vi "HFRR ADV v044.vi"() -> ()   [LabVIEW 2025] (continued)
                "image data" <- w1507
                n1350 = local write "Print 3"(FALSE ("Print 2")) -> ()
                n1351 = call <vilib>:"Draw Flattened Pixmap.vi"("image data"=w1507) -> ("new picture"=→"new picture":picture)  [unwired: 8 in]
              }
              frame Error {
              }
            }
          }
        }
      }
    }
    n1352 = Wait (ms)(milliseconds to wait=u32 20 ("millisecond timer value")) -> ()  [unwired: 1 out]
    n1353 = local read "Quit"() -> (w1440:bool)
  }
  n1354 = while {
    tunnel: w43 -> [_]
    tunnel: w29 -> [_]
    stop <- w1537 stop-if-true
    # "New Adv Logics"
    n1355 = local read "Main Tab"() -> (w1518:T4)
    n1356 = local read "Main Tab"() -> (w1535:T4)
    n1357 = local read "Sign In"() -> (w1534:bool)
    n1358 = case shown="\"Adv Scar\"" w1518 {
      frame "HOME", Default {
        n1359 = local read "LIVE FEED MIN TEMP"() -> (w1670:bool)
        n1360 = local write "LIVE FEED MAX TEMP"(TRUE ("LIVE FEED MAX TEMP")) -> ()
        n1361 = local read "CAMERA ROI MIN TEMP"() -> (w1668:bool)
        n1362 = case shown="True" w1670 {
          selector: w1670 -> [_ w1677]
          frame False {
          }
          frame True {
            n1363 = Not(x=w1677) -> (.not. x?=w1676:bool)
            n1364 = local write "LIVE FEED MIN TEMP"(w1676) -> ()
            n1365 = call "CAMERA LIVE FEED FGV.vi"("Enum - Menu"=CAMERA_LIVE_FEED_ENUM."CAMERA MINIMIZE") -> ()  [unwired: 9 in, 2 out]
          }
        }
        n1366 = case shown="True" w1668 {
          selector: w1668 -> [_ w1674]
          frame False {
          }
          frame True {
            n1367 = Not(x=w1674) -> (.not. x?=w1673:bool)
            n1368 = local write "CAMERA ROI MIN TEMP"(w1673) -> ()
            n1369 = call "IMAGE ANALYSIS.vi"("Enum"=POST_ANALYSIS_ENUM."MINIMIZE UI") -> ()  [unwired: 9 in, 2 out]
          }
        }
        n1370 = local write "CAMERA ROI MAX TEMP"(TRUE ("CAMERA ROI MAX TEMP")) -> ()
      }
      frame "Test Setup" {
        n1371 = local read "LIVE FEED MIN TEMP"() -> (w1680:bool)
        n1372 = local read "CAMERA ROI MIN TEMP"() -> (w1678:bool)
        n1373 = local write "LIVE FEED MAX TEMP"(TRUE ("LIVE FEED MAX TEMP")) -> ()
        n1374 = case shown="True" w1680 {
          selector: w1680 -> [_ w1687]
          frame False {
          }
          frame True {
            n1375 = Not(x=w1687) -> (.not. x?=w1686:bool)
            n1376 = local write "LIVE FEED MIN TEMP"(w1686) -> ()
            n1377 = call "CAMERA LIVE FEED FGV.vi"("Enum - Menu"=CAMERA_LIVE_FEED_ENUM."CAMERA MINIMIZE") -> ()  [unwired: 9 in, 2 out]
          }
        }
        n1378 = case shown="True" w1678 {
          selector: w1678 -> [_ w1684]
          frame False {
          }
          frame True {
            n1379 = Not(x=w1684) -> (.not. x?=w1683:bool)
            n1380 = local write "CAMERA ROI MIN TEMP"(w1683) -> ()
            n1381 = call "IMAGE ANALYSIS.vi"("Enum"=POST_ANALYSIS_ENUM."MINIMIZE UI") -> ()  [unwired: 9 in, 2 out]
          }
        }
        n1382 = local write "CAMERA ROI MAX TEMP"(TRUE ("CAMERA ROI MAX TEMP")) -> ()
      }
      frame "Acquire" {
        n1383 = local read "LIVE FEED MIN TEMP"() -> (w1690:bool)
        n1384 = local write "LIVE FEED MAX TEMP"(TRUE ("LIVE FEED MAX TEMP")) -> ()
        n1385 = local read "CAMERA ROI MIN TEMP"() -> (w1688:bool)
        n1386 = case shown="True" w1690 {
          selector: w1690 -> [_ w1697]
          frame False {
          }
          frame True {
            n1387 = Not(x=w1697) -> (.not. x?=w1696:bool)
            n1388 = local write "LIVE FEED MIN TEMP"(w1696) -> ()
            n1389 = call "CAMERA LIVE FEED FGV.vi"("Enum - Menu"=CAMERA_LIVE_FEED_ENUM."CAMERA MINIMIZE") -> ()  [unwired: 9 in, 2 out]
          }
        }
        n1390 = case shown="True" w1688 {
          selector: w1688 -> [_ w1694]
          frame False {
          }
          frame True {
            n1391 = Not(x=w1694) -> (.not. x?=w1693:bool)
            n1392 = local write "CAMERA ROI MIN TEMP"(w1693) -> ()
            n1393 = call "IMAGE ANALYSIS.vi"("Enum"=POST_ANALYSIS_ENUM."MINIMIZE UI") -> ()  [unwired: 9 in, 2 out]
          }
        }
        n1394 = local write "CAMERA ROI MAX TEMP"(TRUE ("CAMERA ROI MAX TEMP")) -> ()
      }
      frame "Adv Scar" {
        n1395 = local read "CAMERA ROI MIN TEMP"() -> (w1698:bool)
        n1396 = case shown="True" "LIVE FEED MAX TEMP" {
          selector: "LIVE FEED MAX TEMP" -> [_ w1719]
          frame False {
          }
          frame True {
            n1397 = Not(x=w1719) -> (.not. x?=w1718:bool)
            n1398 = local write "LIVE FEED MAX TEMP"(w1718) -> ()
            n1399 = call "CAMERA LIVE FEED FGV.vi"("Enum - Menu"=CAMERA_LIVE_FEED_ENUM."CAMERA RESTORE") -> ("error out"=w1709:errorcluster)  [unwired: 9 in, 1 out]
            n1400 = Type Cast(type=30, x=0) -> (*(type *) &x=w1713:i32)
            n1401 = Add(x=w1713, y=48) -> (x+y=w1714:i32)
            n1402 = call "CAMERA LIVE FEED FGV.vi"("Enum - Menu"=CAMERA_LIVE_FEED_ENUM."CAMERA MODE SET", "error in (no error)"=w1709, "CAMERA MODE"=w1714) -> ("error out"=w1706:errorcluster)  [unwired: 7 in, 1 out]
            n1403 = call "CAMERA LIVE FEED FGV.vi"("Enum - Menu"=CAMERA_LIVE_FEED_ENUM."CAMERA GRAY", "error in (no error)"=w1706) -> ("error out"=w1705:errorcluster)  [unwired: 8 in, 1 out]
            n1404 = call "LIST FILE NAMES.vi"("error in (no error)"=w1705) -> ("error out"=w1715:errorcluster, "filenames"=w1716:string[])  [unwired: 9 in]
            n1405 = property on="FILE 3" class="CmbBox"(error in=w1715, "Strings[]"=w1716) -> ()  [unwired: 1 in, 2 out]
          }
        }
        n1406 = case shown="True" w1698 {
          selector: w1698 -> [_ w1704]
          frame False {
          }
          frame True {
            n1407 = Not(x=w1704) -> (.not. x?=w1703:bool)
            n1408 = local write "CAMERA ROI MIN TEMP"(w1703) -> ()
            n1409 = call "IMAGE ANALYSIS.vi"("Enum"=POST_ANALYSIS_ENUM."MINIMIZE UI") -> ()  [unwired: 9 in, 2 out]
          }
        }
        n1410 = local write "CAMERA ROI MAX TEMP"(TRUE ("CAMERA ROI MAX TEMP")) -> ()
        "LIVE FEED MIN TEMP" <- TRUE ("LIVE FEED MIN TEMP")
      }
      frame "Adv Scar Report" {
        n1411 = local read "CAMERA ROI MAX TEMP"() -> (w1720:bool)
        n1412 = local read "LIVE FEED MIN TEMP"() -> (w1722:bool)
        n1413 = local write "LIVE FEED MAX TEMP"(TRUE ("LIVE FEED MAX TEMP")) -> ()
        n1414 = case shown="True" w1722 {
          selector: w1722 -> [_ w1731]
          frame False {
          }
          frame True {
            n1415 = Not(x=w1731) -> (.not. x?=w1730:bool)
            n1416 = local write "LIVE FEED MIN TEMP"(w1730) -> ()
            n1417 = call "CAMERA LIVE FEED FGV.vi"("Enum - Menu"=CAMERA_LIVE_FEED_ENUM."CAMERA MINIMIZE") -> ()  [unwired: 9 in, 2 out]
          }
        }
        n1418 = case shown="True" w1720 {
          selector: w1720 -> [_ w1728]
          frame False {
          }
          frame True {
            n1419 = Not(x=w1728) -> (.not. x?=w1726:bool)
            n1420 = local write "CAMERA ROI MAX TEMP"(w1726) -> ()
            n1421 = call "IMAGE ANALYSIS.vi"("Enum"=POST_ANALYSIS_ENUM."SHOW UI") -> ("error out"=w1725:errorcluster)  [unwired: 9 in, 1 out]
            n1422 = call "LIST FILE NAMES.vi"("error in (no error)"=w1725) -> ("filenames"=w1724:string[])  [unwired: 9 in, 1 out]
            n1423 = property on="Test File List :" class="CmbBox"("Strings[]"=w1724) -> ()  [unwired: 2 in, 2 out]
          }
        }
        n1424 = local write "CAMERA ROI MIN TEMP"(TRUE ("CAMERA ROI MIN TEMP")) -> ()
      }
      frame "Compare Files" {
        n1425 = local read "LIVE FEED MIN TEMP"() -> (w1734:bool)
        n1426 = local write "LIVE FEED MAX TEMP"(TRUE ("LIVE FEED MAX TEMP")) -> ()
        n1427 = local read "CAMERA ROI MIN TEMP"() -> (w1732:bool)
        n1428 = case shown="True" w1734 {
          selector: w1734 -> [_ w1741]
          frame False {
          }
          frame True {
            n1429 = Not(x=w1741) -> (.not. x?=w1740:bool)
            n1430 = local write "LIVE FEED MIN TEMP"(w1740) -> ()
            n1431 = call "CAMERA LIVE FEED FGV.vi"("Enum - Menu"=CAMERA_LIVE_FEED_ENUM."CAMERA MINIMIZE") -> ()  [unwired: 9 in, 2 out]
          }
        }
        n1432 = case shown="True" w1732 {
          selector: w1732 -> [_ w1738]
          frame False {
          }
          frame True {
            n1433 = Not(x=w1738) -> (.not. x?=w1737:bool)
            n1434 = local write "CAMERA ROI MIN TEMP"(w1737) -> ()
            n1435 = call "IMAGE ANALYSIS.vi"("Enum"=POST_ANALYSIS_ENUM."MINIMIZE UI") -> ()  [unwired: 9 in, 2 out]
          }
        }
        n1436 = local write "CAMERA ROI MAX TEMP"(TRUE ("CAMERA ROI MAX TEMP")) -> ()
      }
      frame "About" {
        n1437 = local read "LIVE FEED MIN TEMP"() -> (w1744:bool)
        n1438 = local write "LIVE FEED MAX TEMP"(TRUE ("LIVE FEED MAX TEMP")) -> ()
        n1439 = local read "CAMERA ROI MIN TEMP"() -> (w1743:bool)
        n1440 = case shown="True" w1744 {
          selector: w1744 -> [_ w1751]
          frame False {
          }
          frame True {
            n1441 = Not(x=w1751) -> (.not. x?=w1750:bool)
            n1442 = local write "LIVE FEED MIN TEMP"(w1750) -> ()
            n1443 = call "CAMERA LIVE FEED FGV.vi"("Enum - Menu"=CAMERA_LIVE_FEED_ENUM."CAMERA MINIMIZE") -> ()  [unwired: 9 in, 2 out]
          }
        }
        n1444 = case shown="True" w1743 {
          selector: w1743 -> [_ w1748]
          frame False {
          }
          frame True {
            n1445 = Not(x=w1748) -> (.not. x?=w1747:bool)
            n1446 = local write "CAMERA ROI MIN TEMP"(w1747) -> ()
            n1447 = call "IMAGE ANALYSIS.vi"("Enum"=POST_ANALYSIS_ENUM."MINIMIZE UI") -> ()  [unwired: 9 in, 2 out]
          }
        }
        n1448 = local write "CAMERA ROI MAX TEMP"(TRUE ("CAMERA ROI MIN TEMP")) -> ()
      }
      frame "Advance" {
        n1449 = local read "LIVE FEED MIN TEMP"() -> (w1754:bool)
        n1450 = local write "LIVE FEED MAX TEMP"(TRUE ("LIVE FEED MAX TEMP")) -> ()
        n1451 = local read "CAMERA ROI MIN TEMP"() -> (w1752:bool)
        n1452 = case shown="True" w1754 {
          selector: w1754 -> [_ w1761]
          frame False {
          }
          frame True {
            n1453 = Not(x=w1761) -> (.not. x?=w1760:bool)
            n1454 = local write "LIVE FEED MIN TEMP"(w1760) -> ()
            n1455 = call "CAMERA LIVE FEED FGV.vi"("Enum - Menu"=CAMERA_LIVE_FEED_ENUM."CAMERA MINIMIZE") -> ()  [unwired: 9 in, 2 out]
          }
        }
        n1456 = local write "CAMERA ROI MAX TEMP"(TRUE ("CAMERA ROI MAX TEMP")) -> ()
        n1457 = case shown="True" w1752 {
          selector: w1752 -> [_ w1758]
          frame False {
          }
          frame True {
            n1458 = Not(x=w1758) -> (.not. x?=w1757:bool)
            n1459 = local write "CAMERA ROI MIN TEMP"(w1757) -> ()
            n1460 = call "IMAGE ANALYSIS.vi"("Enum"=POST_ANALYSIS_ENUM."MINIMIZE UI") -> ()  [unwired: 9 in, 2 out]
          }
        }
      }
      frame "Mooha" {
        n1461 = local read "LIVE FEED MIN TEMP"() -> (w1764:bool)
        n1462 = local write "LIVE FEED MAX TEMP"(TRUE ("LIVE FEED MAX TEMP")) -> ()
        n1463 = local read "CAMERA ROI MIN TEMP"() -> (w1762:bool)
        n1464 = case shown="True" w1764 {
          selector: w1764 -> [_ w1771]
          frame False {
          }
          frame True {
            n1465 = Not(x=w1771) -> (.not. x?=w1770:bool)
            n1466 = local write "LIVE FEED MIN TEMP"(w1770) -> ()
            n1467 = call "CAMERA LIVE FEED FGV.vi"("Enum - Menu"=CAMERA_LIVE_FEED_ENUM."CAMERA MINIMIZE") -> ()  [unwired: 9 in, 2 out]
          }
        }
        n1468 = local write "CAMERA ROI MAX TEMP"(TRUE ("CAMERA ROI MAX TEMP")) -> ()
        n1469 = case shown="True" w1762 {
          selector: w1762 -> [_ w1768]
          frame False {
          }
          frame True {
            n1470 = Not(x=w1768) -> (.not. x?=w1767:bool)
            n1471 = local write "CAMERA ROI MIN TEMP"(w1767) -> ()
            n1472 = call "IMAGE ANALYSIS.vi"("Enum"=POST_ANALYSIS_ENUM."MINIMIZE UI") -> ()  [unwired: 9 in, 2 out]
          }
        }
      }
    }
    n1473 = local read "Auto Start Test"() -> (w1509:bool)
    n1474 = case shown="True" "sign in temp" {
      frame False {
      }
      frame True {
        w1544 = 1 ("y")
        n1475 = local read "USERNAME"() -> (w1550:string)
        n1476 = local read "USER ID"() -> (w1547:string)
        n1477 = call <vilib>:"Trim Whitespace.vi"("string"=w1550) -> ("trimmed string"=w1549:string)  [unwired: 1 in]
        n1478 = call <vilib>:"Trim Whitespace.vi"("string"=w1547) -> ("trimmed string"=w1548:string)  [unwired: 1 in]
        n1479 = String Length(string=w1549) -> (length=w1546:i32)
        n1480 = String Length(string=w1548) -> (length=w1545:i32)
        n1481 = Greater?(x=w1546, y=w1544) -> (0:w1543:bool)
        n1482 = Greater?(x=w1545, y=w1544) -> (0:w1542:bool)
        n1483 = And(x=w1543, y=w1542) -> (x .and. y?=w1541:bool)
        n1484 = case shown="True" w1541 {
          frame False {
            n1485 = property on="Sign In" class="Bool (strict)"("DisabledEnum"=T19."Disabled" ("Disabled")) -> ()  [unwired: 2 in, 2 out]
          }
          frame True {
            n1486 = property on="Sign In" class="Bool (strict)"("DisabledEnum"=T19."Enabled" ("Disabled")) -> ()  [unwired: 2 in, 2 out]
          }
        }
      }
    }
    n1487 = local read "Air Temperature"() -> (w1526:bool)
    n1488 = local read "Coefficient Of Friction"() -> (w1527:bool)
    n1489 = case shown="False" w1509 {
      frame False {
        n1490 = local read "Auto stop temp"() -> (w1538:bool)
        n1491 = case shown="True" w1538 {
          frame False {
          }
          frame True {
            n1492 = local write "Auto Start Temp"(FALSE ("Auto Start Temp")) -> ()
          }
        }
      }
      frame True {
        "Auto stop temp" <- TRUE ("Auto stop temp")
      }
    }
    n1493 = local read "Humidity 3"() -> (w1525:bool)
    n1494 = case shown="\"HOME\"" w1535 {
      frame "HOME" {
        n1495 = local write "main tab sub"(enum32{"Page 1", "Page 2"}."Page 1" ("main tab sub")) -> ()
      }
      frame Default {
        n1496 = local write "main tab sub"(enum32{"Page 1", "Page 2"}."Page 2" ("main tab sub")) -> ()
      }
    }
    n1497 = case shown="True" w1534 {
      selector: w1534 -> [_ w1886]
      frame False {
      }
      frame True {
        n1498 = Not(x=w1886) -> (.not. x?=w1885:bool)
        n1499 = local write "Sign In"(w1885) -> ()
        n1500 = local write "Main Dashboard Buttons"(T25."Test Setup" ("Main Dashboard Buttons")) -> ()
      }
    }
    n1501 = case shown="\"Numeric Display\", Default" "Num/Graph" {
      frame "Numeric Display", Default {
        n1502 = property on="Single/Multiple" class="RadioBtnsControl (strict)"("Visible"=FALSE) -> ()  [unwired: 2 in, 2 out]
        n1503 = property on="Single - Graph" class="Ring (strict)"("Visible"=FALSE) -> ()  [unwired: 2 in, 2 out]
        n1504 = local write "Main Tab Display"(T6."Dashboard 1" ("Main Tab Display")) -> ()
      }
      frame "Graph Display" {
        n1505 = property on="Single/Multiple" class="RadioBtnsControl (strict)"("Visible"=TRUE) -> ()  [unwired: 2 in, 2 out]
        n1506 = case shown="\"Multiple\"" "Single/Multiple" {
          frame "Single ", Default {
            n1507 = property on="Single - Graph" class="Ring (strict)"("Visible"=TRUE) -> ()  [unwired: 2 in, 2 out]
            n1508 = local write "Main Tab Display"(T6."Dashboard 3" ("Main Tab Display")) -> ()
          }
          frame "Multiple" {
            n1509 = property on="Single - Graph" class="Ring (strict)"("Visible"=FALSE) -> ()  [unwired: 2 in, 2 out]
            n1510 = local write "Main Tab Display"(T6."Dashboard 2" ("Main Tab Display")) -> ()
          }
        }
      }
    }
    n1511 = local read "Stroke"() -> (w1524:bool)
    n1512 = local read "USERNAME"() -> (w1529:string)
    n1513 = case shown="True" w1527 {
      selector: w1527 -> [_ w1811]
      frame False {
      }
      frame True {
        n1514 = Not(x=w1811) -> (.not. x?=w1810:bool)
        n1515 = local write "Coefficient Of Friction"(w1810) -> ()
        n1516 = local write "Tab Control 2"(T8."Coefficient Of Friction" ("Tab Control 2")) -> ()
      }
    }
    n1517 = case shown="True" w1526 {
      selector: w1526 -> [_ w1808]
      frame False {
      }
      frame True {
        n1518 = Not(x=w1808) -> (.not. x?=w1806:bool)
        n1519 = local write "Air Temperature"(w1806) -> ()
        n1520 = local write "Tab Control 2"(T8."Air Temperature" ("Tab Control 2")) -> ()
      }
    }
    n1521 = case shown="True" w1524 {
      selector: w1524 -> [_ w1802]
      frame False {
      }
      frame True {
        n1522 = Not(x=w1802) -> (.not. x?=w1800:bool)
        n1523 = local write "Stroke"(w1800) -> ()
        n1524 = local write "Tab Control 2"(T8."Stroke" ("Tab Control 2")) -> ()
      }
    }
    n1525 = local write "tested by"(w1529) -> ()
    n1526 = case shown="True" w1525 {
      selector: w1525 -> [_ w1805]
      frame False {
      }
      frame True {
        n1527 = Not(x=w1805) -> (.not. x?=w1803:bool)
        n1528 = local write "Humidity 3"(w1803) -> ()
        n1529 = local write "Tab Control 2"(T8."Humidity" ("Tab Control 2")) -> ()
      }
    }
    n1530 = case shown="\"Calibration\"" "Main Dashboard Buttons" {
      tunnel: [T4."HOME" ("Main Tab") T4."Test Setup" ("Main Tab") T4."Acquire" ("Main Tab") T4."Adv Scar" ("Main Tab") T4."Adv Scar Report" ("Main Tab") T4."Compare Files" ("Main Tab") T4."Calibration" ("Main Tab") T4."About" ("Main Tab") T4."Advance" ("Main Tab")] -> w1508
      frame "Home", Default {
      }
      frame "Test Setup" {
      }
      frame "Dashboard" {
      }
      frame "Imaging" {
      }
      frame "Report" {
      }
      frame "Analysis" {
      }
      frame "Calibration" {
      }
      frame "About" {
      }
      frame "Advance" {
      }
    }
    n1531 = Wait (ms)(milliseconds to wait=u32 100) -> ()  [unwired: 1 out]
    n1532 = local read "Main Tab Display"() -> (w1528:T6)
    n1533 = local write "Main Tab"(w1508) -> ()
    n1534 = case shown="\"Dashboard 3\"" w1528 {
      frame "Dashboard 1", Default {
        n1535 = property on="Reset Graph" class="Bool (strict)"("Visible"=FALSE) -> ()  [unwired: 2 in, 2 out]
      }
      frame "Dashboard 2" {
        n1536 = property on="Reset Graph" class="Bool (strict)"("Visible"=TRUE) -> ()  [unwired: 2 in, 2 out]
      }
      frame "Dashboard 3" {
        n1537 = property on="Reset Graph" class="Bool (strict)"("Visible"=TRUE) -> ()  [unwired: 2 in, 2 out]
      }
    }
    n1538 = local read "SCAR MEASURMENT"() -> (w1516:enum32{"Auto Scar", "Manual Scar"})
    n1539 = local read "Humidity"() -> (w1530:bool)
    n1540 = local read "Cap Live Image"() -> (w1513:bool)
    n1541 = local read "Sample Temperature"() -> (w1523:bool)
    n1542 = local read "Air Temp vs Humidity"() -> (w1521:bool)
    n1543 = local read "Frequency"() -> (w1522:bool)
    n1544 = case shown="False" w1530 {
      frame False {
        n1545 = local write "Humidity On Command"(TRUE ("Humidity On Command")) -> ()
        n1546 = case shown="True" "Humidity Off Command" {
          selector: "Humidity Off Command" -> [_ w1818]
          frame False {
          }
          frame True {
            n1547 = stacked-sequence {
              frame #0 {
                n1548 = local read "WriteHumidity"() -> (w1820:string[])
                n1549 = Insert Into Array(array=w1820, new element="R;1" ("new element/subarray")) -> (w1819:string[])  [unwired: 1 in]
                n1550 = local write "WriteHumidity"(w1819) -> ()
              }
              frame #1 {
                n1551 = Wait (ms)(milliseconds to wait=u32 500) -> ()  [unwired: 1 out]
              }
              frame #2 {
                n1552 = local read "WriteHumidity"() -> (w1824:string[])
                n1553 = local read "EVENT LOG"() -> (w1828:string)
                n1554 = call "Event Log.vi"("Content"="Humidity Control Off" ("string"), "EVENT LOG"=w1828) -> ("EVENT LOG"=w1829:string)  [unwired: 8 in, 1 out]
                n1555 = local write "EVENT LOG"(w1829) -> ()
                n1556 = Insert Into Array(array=w1824, new element="R;1" ("new element/subarray")) -> (w1825:string[])  [unwired: 1 in]
                n1557 = local write "WriteHumidity"(w1825) -> ()
                n1558 = local write "Humidity 2"(TRUE ("Humidity")) -> ()
              }
            }
            n1559 = Not(x=w1818) -> (.not. x?=w1817:bool)
            n1560 = local write "Humidity Off Command"(w1817) -> ()
          }
        }
      }
      frame True {
        n1561 = local write "Humidity Off Command"(TRUE ("Humidity Off Command")) -> ()
        n1562 = case shown="False" "Humidity On Command" {
          selector: "Humidity On Command" -> [_ w1833]
          frame False {
          }
          frame True {
            n1563 = stacked-sequence {
              frame #0 {
                n1564 = local read "Set Rh"() -> (w1839:dbl)
                n1565 = local read "WriteHumidity"() -> (w1835:string[])
                n1566 = Number To Fractional String(number=w1839, precision (6)=i16 2) -> (F-format string=w1840:string)  [unwired: 2 in]
                n1567 = Concatenate Strings("M;" ("new element/subarray"), w1840) -> (w1838:string)
                n1568 = Insert Into Array(array=w1835, new element=w1838) -> (w1834:string[])  [unwired: 1 in]
                n1569 = local write "WriteHumidity"(w1834) -> ()
              }
              frame #1 {
                n1570 = Wait (ms)(milliseconds to wait=u32 500) -> ()  [unwired: 1 out]
              }
              frame #2 {
                n1571 = local read "WriteHumidity"() -> (w1843:string[])
                n1572 = local read "Set Rh"() -> (w1847:dbl)
                n1573 = Number To Fractional String(number=w1847, precision (6)=i16 2) -> (F-format string=w1848:string)  [unwired: 2 in]
                n1574 = Concatenate Strings("M;" ("new element/subarray"), w1848) -> (w1846:string)
                n1575 = Insert Into Array(array=w1843, new element=w1846) -> (w1842:string[])  [unwired: 1 in]
                n1576 = local write "WriteHumidity"(w1842) -> ()
              }
              frame #3 {
                n1577 = Wait (ms)(milliseconds to wait=u32 500) -> ()  [unwired: 1 out]
              }
              frame #4 {
                (unwired) "% RH" ("string")
                (unwired) i16 2 ("precision (6)")
                (unwired) "M;" ("new element/subarray")
                n1578 = local read "Set Rh"() -> (w1857:dbl)
                n1579 = local read "WriteHumidity"() -> (w1850:string[])
                n1580 = Number To Fractional String(number=w1857, precision (6)=i16 2) -> (F-format string=w1854:string)  [unwired: 2 in]
                n1581 = Concatenate Strings("M;" ("new element/subarray"), w1854) -> (w1858:string)
                n1582 = Concatenate Strings("Humidity Set to : " ("string"), w1854, "% RH" ("string")) -> (w1852:string)
                n1583 = Insert Into Array(array=w1850, new element=w1858) -> (w1851:string[])  [unwired: 1 in]
                n1584 = disable-structure shown="Enabled" {
                  frame Enabled {
                    n1585 = local read "EVENT LOG"() -> (w1861:string)
                    n1586 = call "Event Log.vi"("Content"="Humidity Control On", "EVENT LOG"=w1861) -> ("EVENT LOG"=w1862:string)  [unwired: 8 in, 1 out]
                    n1587 = local write "EVENT LOG"(w1862) -> ()
                  }
                  frame Disabled {
                  }
                }
                n1588 = disable-structure shown="Enabled" {
                  disable-tunnel: w1852 -> [_ _]
                  frame Enabled {
                    n1589 = local read "EVENT LOG"() -> (w1864:string)
                    n1590 = call "Event Log.vi"("Content"="Humidity Control On", "EVENT LOG"=w1864) -> ("EVENT LOG"=w1865:string)  [unwired: 8 in, 1 out]
                    n1591 = local write "EVENT LOG"(w1865) -> ()
                  }
                  frame Disabled {
                  }
                }
                n1592 = local write "WriteHumidity"(w1851) -> ()
              }
            }
            n1593 = Not(x=w1833) -> (.not. x?=w1832:bool)
            n1594 = local write "Humidity On Command"(w1832) -> ()
          }
        }
      }
    }
    n1595 = Equal?(x=w1516, y=enum32{"Auto Scar", "Manual Scar"}."Auto Scar" ("SCAR MEASURMENT")) -> (x = y?=w1512:bool)
    n1596 = local read "TEST STANDARD"() -> (w1519:T5)
    n1597 = And(x=w1513, y=w1512) -> (x .and. y?=w1514:bool)
    n1598 = case shown="True" w1514 {
      selector: w1514 -> [_ w1617]
      tunnel: errorcluster {"status"=FALSE, "code"=0, "source"=""} ("error in (no error) 3") -> [_ w1618]
      frame False {
      }
      frame True {
        n1599 = stacked-sequence {
          tunnel: w1618 -> [_ _ _ _ _ _ _ w1666]
          tunnel: w1617 -> [_ _ _ _ _ w1647 _ _]
          frame #0 {
            n1600 = call "CAMERA LIVE FEED FGV.vi"("Enum - Menu"=CAMERA_LIVE_FEED_ENUM."CAMERA MINIMIZE") -> ()  [unwired: 9 in, 2 out]
          }
          frame #1 {
            n1601 = property on="Auto Scar Check  2" class="Clust (strict)"("Visible"=TRUE) -> ()  [unwired: 2 in, 2 out]
          }
          frame #2 {
            n1602 = String To Path(string="C:\\LAB-IQ\\Image Calibrate v01.dcf") -> (path=w1623:path)
            n1603 = Open/Create/Replace File ("Open File")(file path (use dialog)=w1623) -> (refnum out=w1624:refnum<file>)  [unwired: 5 in, 2 out]
            n1604 = for {
              N: 4 -> [_]
              tunnel: w1624 -> [w1630]
              i -> [w1626]
              n1605 = Read from Text File ("Read File")(file (use dialog)=w1630) -> (text=w1631:string)  [unwired: 3 in, 3 out]
              n1606 = String Subset(string=w1631, offset (0)=6, length (rest)=10 ("length (rest)")) -> (substring=w1627:string)
              n1607 = Fract/Exp String To Number(string=w1627) -> (number=w1625:dbl)  [unwired: 3 in, 1 out]
              n1608 = case shown="0" w1626 {
                tunnel: w1625 -> [w1632 w1633 _ w1634 _]
                frame 0 {
                  "5x Gain" <- w1632
                }
                frame 1 {
                  "10x Gain" <- w1633
                }
                frame 2 {
                }
                frame 3 {
                  "100x gain" <- w1634
                }
                frame 4, Default {
                }
              }
            }
          }
          frame #3 {
            n1609 = local read "FILE 3"() -> (w1640:string)
            n1610 = call <vilib>:"Trim Whitespace.vi"("string"="C:\\LAB-IQ\\images\\") -> ("trimmed string"=w1642:string)  [unwired: 1 in]
            n1611 = String To Path(string=w1642) -> (path=w1641:path)
            n1612 = Concatenate Strings(w1640, ".png" ("string")) -> (w1639:string)
            n1613 = Build Path(base path=w1641, name or relative path=w1639) -> (appended path=w1637:path)
            "Image path" <- w1637
            n1614 = Path To String(path=w1637) -> (string=w1636:string)
            n1615 = call "CAMERA LIVE FEED FGV.vi"("Enum - Menu"=CAMERA_LIVE_FEED_ENUM."CAMERA SAVE", "Image Path"=w1636) -> ()  [unwired: 8 in, 2 out]
          }
          frame #4 {
            n1616 = One Button Dialog(message="Image saved successfully") -> ()  [unwired: 1 in, 1 out]
          }
          frame #5 {
            n1617 = local read "TEST STANDARD"() -> (w1646:T5)
            n1618 = local read "Magnification len live scar"() -> (w1658:string)
            n1619 = Not(x=w1647) -> (.not. x?=w1648:bool)
            n1620 = local write "Cap Live Image"(w1648) -> ()
            n1621 = case shown="\"ISO 12156\"" w1646 {
              tunnel: ["ASTM D6079" "ISO 12156"] -> w1645
              frame "ASTM D6079", Default {
              }
              frame "ISO 12156" {
              }
            }
            n1622 = case shown="\"5x\", Default" w1658 {
              tunnel: [w1661 w1662] -> w1657
              frame "5x", Default {
                n1623 = local read "5x Gain"() -> (w1661:dbl)
              }
              frame "10x" {
                # "5x"
                n1624 = local read "10x Gain"() -> (w1662:dbl)
              }
            }
            n1625 = local read "Image path"() -> (w1656:path)
            n1626 = local read "FILE 3"() -> (w1649:string)
            n1627 = call "EDGE DETCTION.vi"("GAIN VALUE"=w1657, "Image Path"=w1656) -> ("error out"=w1655:errorcluster, "return value"=w1654:cluster{string, string, dbl, dbl, dbl})  [unwired: 8 in]
            n1628 = Bundle By Name(cluster=T26 {"File Name"="", "Test Method"="", "Operator"="", "Fuel Description"="", "Date and time"=""} ("Main Ref"), "File Name"=w1649, "Test Method"=w1645) -> (w1650:T26)
            n1629 = call "duf file read.vi"("error in (no error)"=w1655, "Main Ref"=w1650) -> ("error out"=w1653:errorcluster, "Main Ref 2"=w1651:T26)  [unwired: 8 in]
            n1630 = call "EDGE DETECTION REPORT.vi"("error in (no error)"=w1653, "return value 2"=w1654, "Main Ref"=w1651) -> ()  [unwired: 8 in, 1 out]
          }
          frame #6 {
            n1631 = property on="Auto Scar Check  2" class="Clust (strict)"("Visible"=FALSE) -> ()  [unwired: 2 in, 2 out]
          }
          frame #7 {
            n1632 = call "CAMERA LIVE FEED FGV.vi"("Enum - Menu"=CAMERA_LIVE_FEED_ENUM."CAMERA MINIMIZE", "error in (no error)"=w1666) -> ()  [unwired: 8 in, 2 out]
            n1633 = local write "Main Dashboard Buttons"(T1."Home" ("Main Dashboard Buttons")) -> ()
            n1634 = local write "Main Tab"(T4."HOME" ("Main Tab")) -> ()
          }
        }
      }
    }
    n1635 = local read "Heater Button"() -> (w1520:bool)
    n1636 = case shown="True" w1522 {
      selector: w1522 -> [_ w1796]
      frame False {
      }
      frame True {
        n1637 = Not(x=w1796) -> (.not. x?=w1794:bool)
        n1638 = local write "Frequency"(w1794) -> ()
        n1639 = local write "Tab Control 2"(T8."Frequency" ("Tab Control 2")) -> ()
      }
    }
    n1640 = case shown="True" w1521 {
      selector: w1521 -> [_ w1793]
      frame False {
      }
      frame True {
        n1641 = Not(x=w1793) -> (.not. x?=w1791:bool)
        n1642 = local write "Air Temp vs Humidity"(w1791) -> ()
        n1643 = local write "Tab Control 2"(T8."Air Temp vs Rh" ("Tab Control 2")) -> ()
      }
    }
    n1644 = case shown="True" w1523 {
      selector: w1523 -> [_ w1799]
      frame False {
      }
      frame True {
        n1645 = Not(x=w1799) -> (.not. x?=w1797:bool)
        n1646 = local write "Sample Temperature"(w1797) -> ()
        n1647 = local write "Tab Control 2"(T8."Sample Temperature" ("Tab Control 2")) -> ()
      }
    }
    n1648 = case shown="\"Custom\"" w1519 {
      frame "ASTM D6079", Default {
        w1772 = "ASTM D6079 TEST CONDITIONS" ("Standard 2")
        n1649 = local write "Standard 2"(w1772) -> ()
        n1650 = local write "Standard"(w1772) -> ()
      }
      frame "ISO 12156" {
        w1773 = "ISO 12156 TEST CONDITIONS" ("Standard 2")
        n1651 = local write "Standard 2"(w1773) -> ()
        n1652 = local write "Standard"(w1773) -> ()
      }
      frame "CEC F-096-A-06" {
        w1774 = "CEC F-096-A-06 TEST CONDITIONS" ("Standard 2")
        n1653 = local write "Standard 2"(w1774) -> ()
        n1654 = local write "Standard"(w1774) -> ()
      }
      frame "Custom" {
        w1775 = "CUSTOM TEST CONDITIONS" ("Standard 2")
        n1655 = local write "Standard 2"(w1775) -> ()
        n1656 = local write "Standard"(w1775) -> ()
      }
    }
    n1657 = case shown="True" w1520 {
      frame False {
        n1658 = local write "Temperature On Command"(TRUE ("Temperature On Command")) -> ()
        n1659 = case shown="True" "Temperature Off Command" {
          selector: "Temperature Off Command" -> [_ w1779]
          frame False {
          }
          frame True {
            n1660 = Not(x=w1779) -> (.not. x?=w1778:bool)
            n1661 = local read "EVENT LOG"() -> (w1782:string)
            n1662 = local write "Temperature Off Command"(w1778) -> ()
            n1663 = call "Event Log.vi"("Content"="Heater Off", "EVENT LOG"=w1782) -> ("EVENT LOG"=w1781:string)  [unwired: 8 in, 1 out]
            n1664 = local write "EVENT LOG"(w1781) -> ()
          }
        }
      }
      frame True {
        n1665 = local write "Temperature Off Command"(TRUE ("Temperature Off Command")) -> ()
        n1666 = case shown="True" "Temperature On Command" {
          selector: "Temperature On Command" -> [_ w1786]
          frame False {
          }
          frame True {
            n1667 = Not(x=w1786) -> (.not. x?=w1785:bool)
            n1668 = local write "Temperature On Command"(w1785) -> ()
            n1669 = disable-structure shown="Enabled" {
              disable-tunnel: "Heater On" -> [w1788 _]
              frame Enabled {
                n1670 = local read "EVENT LOG"() -> (w1789:string)
                n1671 = call "Event Log.vi"("Content"=w1788, "EVENT LOG"=w1789) -> ("EVENT LOG"=w1790:string)  [unwired: 8 in, 1 out]
                n1672 = local write "EVENT LOG"(w1790) -> ()
              }
              frame Disabled {
              }
            }
          }
        }
      }
    }
    n1673 = local read "Main Tab"() -> (w1511:T4)
    n1674 = case shown="\"About\"" w1511 {
      frame "HOME", Default {
        w1553 = T19."Enabled" ("Disabled")
        n1675 = local read "Service Password enable"() -> (w1555:bool)
        n1676 = property on="Imaging" class="Bool (strict)"("DisabledEnum"=w1553) -> ()  [unwired: 2 in, 2 out]
        n1677 = property on="Dashboard" class="Bool (strict)"("DisabledEnum"=w1553) -> ()  [unwired: 2 in, 2 out]
        n1678 = property on="Test Setup" class="Bool (strict)"("DisabledEnum"=w1553) -> ()  [unwired: 2 in, 2 out]
        n1679 = property on="Analysis" class="Bool (strict)"("DisabledEnum"=w1553) -> ()  [unwired: 2 in, 2 out]
        n1680 = property on="Home" class="Bool (strict)"("DisabledEnum"=w1553) -> ()  [unwired: 2 in, 2 out]
        n1681 = property on="Report" class="Bool (strict)"("DisabledEnum"=w1553) -> ()  [unwired: 2 in, 2 out]
        n1682 = property on="Main Dashboard Buttons" class="RadioBtnsControl (strict)"("DisabledEnum"=w1553) -> ()  [unwired: 2 in, 2 out]
        n1683 = property on="Calibration" class="Bool (strict)"("DisabledEnum"=w1553) -> ()  [unwired: 2 in, 2 out]
        n1684 = case shown="True" w1555 {
          tunnel: [T19."Disabled" ("Disabled") T19."Enabled" ("Disabled")] -> w1554
          frame False {
          }
          frame True {
          }
        }
        n1685 = property on="About" class="Bool (strict)"("DisabledEnum"=w1554) -> ()  [unwired: 2 in, 2 out]
      }
      frame "Test Setup" {
        w1560 = T19."Enabled" ("Disabled")
        n1686 = local read "Service Password enable"() -> (w1559:bool)
        n1687 = property on="Dashboard" class="Bool (strict)"("DisabledEnum"=T19."Disabled" ("Disabled")) -> ()  [unwired: 2 in, 2 out]
        n1688 = property on="Imaging" class="Bool (strict)"("DisabledEnum"=w1560) -> ()  [unwired: 2 in, 2 out]
        n1689 = property on="Analysis" class="Bool (strict)"("DisabledEnum"=w1560) -> ()  [unwired: 2 in, 2 out]
        n1690 = property on="Home" class="Bool (strict)"("DisabledEnum"=w1560) -> ()  [unwired: 2 in, 2 out]
        n1691 = property on="Report" class="Bool (strict)"("DisabledEnum"=w1560) -> ()  [unwired: 2 in, 2 out]
        n1692 = property on="Test Setup" class="Bool (strict)"("DisabledEnum"=w1560) -> ()  [unwired: 2 in, 2 out]
        n1693 = case shown="True" w1559 {
          tunnel: [T19."Disabled" ("Disabled") T19."Enabled" ("Disabled")] -> w1558
          frame False {
          }
          frame True {
          }
        }
        n1694 = property on="About" class="Bool (strict)"("DisabledEnum"=w1558) -> ()  [unwired: 2 in, 2 out]
      }
      frame "Adv Scar" {
        w1567 = T19."Enabled" ("Disabled")
        n1695 = property on="Dashboard" class="Bool (strict)"("DisabledEnum"=T19."Disabled" ("Disabled")) -> ()  [unwired: 2 in, 2 out]
        n1696 = property on="Imaging" class="Bool (strict)"("DisabledEnum"=w1567) -> ()  [unwired: 2 in, 2 out]
        n1697 = property on="Analysis" class="Bool (strict)"("DisabledEnum"=w1567) -> ()  [unwired: 2 in, 2 out]
        n1698 = property on="Home" class="Bool (strict)"("DisabledEnum"=w1567) -> ()  [unwired: 2 in, 2 out]
        n1699 = property on="Report" class="Bool (strict)"("DisabledEnum"=w1567) -> ()  [unwired: 2 in, 2 out]
        n1700 = property on="Test Setup" class="Bool (strict)"("DisabledEnum"=w1567) -> ()  [unwired: 2 in, 2 out]
        n1701 = local read "Service Password enable"() -> (w1565:bool)
        n1702 = case shown="True" w1565 {
          tunnel: [T19."Disabled" ("Disabled") T19."Enabled" ("Disabled")] -> w1564
          frame False {
          }
          frame True {
          }
        }
        n1703 = property on="About" class="Bool (strict)"("DisabledEnum"=w1564) -> ()  [unwired: 2 in, 2 out]
      }
      frame "Calibration" {
        w1570 = T19."Enabled" ("Disabled")
        n1704 = property on="Dashboard" class="Bool (strict)"("DisabledEnum"=T19."Disabled" ("Disabled")) -> ()  [unwired: 2 in, 2 out]
        n1705 = property on="Imaging" class="Bool (strict)"("DisabledEnum"=w1570) -> ()  [unwired: 2 in, 2 out]
        n1706 = property on="Analysis" class="Bool (strict)"("DisabledEnum"=w1570) -> ()  [unwired: 2 in, 2 out]
        n1707 = property on="Home" class="Bool (strict)"("DisabledEnum"=w1570) -> ()  [unwired: 2 in, 2 out]
        n1708 = property on="Report" class="Bool (strict)"("DisabledEnum"=w1570) -> ()  [unwired: 2 in, 2 out]
        n1709 = property on="Test Setup" class="Bool (strict)"("DisabledEnum"=w1570) -> ()  [unwired: 2 in, 2 out]
        n1710 = local read "Service Password enable"() -> (w1572:bool)
        n1711 = property on="Calibration" class="Bool (strict)"("DisabledEnum"=w1570) -> ()  [unwired: 2 in, 2 out]
        n1712 = case shown="True" w1572 {
          tunnel: [T19."Disabled" ("Disabled") T19."Enabled" ("Disabled")] -> w1571
          frame False {
          }
          frame True {
          }
        }
        n1713 = property on="About" class="Bool (strict)"("DisabledEnum"=w1571) -> ()  [unwired: 2 in, 2 out]
      }
      frame "Adv Scar Report" {
        w1578 = T19."Enabled" ("Disabled")
        n1714 = property on="Dashboard" class="Bool (strict)"("DisabledEnum"=T19."Disabled" ("Disabled")) -> ()  [unwired: 2 in, 2 out]
        n1715 = property on="Imaging" class="Bool (strict)"("DisabledEnum"=w1578) -> ()  [unwired: 2 in, 2 out]
        n1716 = property on="Analysis" class="Bool (strict)"("DisabledEnum"=w1578) -> ()  [unwired: 2 in, 2 out]
        n1717 = property on="Home" class="Bool (strict)"("DisabledEnum"=w1578) -> ()  [unwired: 2 in, 2 out]
        n1718 = property on="Report" class="Bool (strict)"("DisabledEnum"=w1578) -> ()  [unwired: 2 in, 2 out]
        n1719 = property on="Test Setup" class="Bool (strict)"("DisabledEnum"=w1578) -> ()  [unwired: 2 in, 2 out]
        n1720 = local read "Service Password enable"() -> (w1577:bool)
        n1721 = case shown="True" w1577 {
          tunnel: [T19."Disabled" ("Disabled") T19."Enabled" ("Disabled")] -> w1576
          frame False {
          }
          frame True {
          }
        }
        n1722 = property on="About" class="Bool (strict)"("DisabledEnum"=w1576) -> ()  [unwired: 2 in, 2 out]
      }
      frame "Compare Files" {
        w1584 = T19."Enabled" ("Disabled")
        n1723 = local read "Service Password enable"() -> (w1583:bool)
        n1724 = property on="Dashboard" class="Bool (strict)"("DisabledEnum"=T19."Disabled" ("Disabled")) -> ()  [unwired: 2 in, 2 out]
        n1725 = property on="Imaging" class="Bool (strict)"("DisabledEnum"=w1584) -> ()  [unwired: 2 in, 2 out]
        n1726 = property on="Analysis" class="Bool (strict)"("DisabledEnum"=w1584) -> ()  [unwired: 2 in, 2 out]
        n1727 = property on="Home" class="Bool (strict)"("DisabledEnum"=w1584) -> ()  [unwired: 2 in, 2 out]
        n1728 = property on="Report" class="Bool (strict)"("DisabledEnum"=w1584) -> ()  [unwired: 2 in, 2 out]
        n1729 = property on="Test Setup" class="Bool (strict)"("DisabledEnum"=w1584) -> ()  [unwired: 2 in, 2 out]
        n1730 = case shown="True" w1583 {
          tunnel: [T19."Disabled" ("Disabled") T19."Enabled" ("Disabled")] -> w1582
          frame False {
          }
          frame True {
          }
        }
        n1731 = property on="About" class="Bool (strict)"("DisabledEnum"=w1582) -> ()  [unwired: 2 in, 2 out]
      }
      frame "Acquire" {
        n1732 = local read "Service Password enable"() -> (w1589:bool)
        n1733 = property on="Test Setup" class="Bool (strict)"("DisabledEnum"=T19."Disabled" ("Disabled")) -> ()  [unwired: 2 in, 2 out]
        n1734 = local read "Auto Start Test"() -> (w1591:bool)
        n1735 = local read "RUN"() -> (w1593:bool)
        n1736 = case shown="True" w1589 {
          tunnel: [T19."Disabled" ("Disabled") T19."Enabled" ("Disabled")] -> w1590
          frame False {
          }
          frame True {
          }
        }
        n1737 = Or(x=w1593, y=w1591) -> (x .or. y?=w1592:bool)
        n1738 = case shown="True" w1592 {
          tunnel: [T19."Enabled" ("Disabled") T19."Disabled" ("Disabled")] -> w1588
          frame False {
          }
          frame True {
          }
        }
        n1739 = property on="About" class="Bool (strict)"("DisabledEnum"=w1590) -> ()  [unwired: 2 in, 2 out]
        n1740 = property on="Imaging" class="Bool (strict)"("DisabledEnum"=w1588) -> ()  [unwired: 2 in, 2 out]
        n1741 = property on="Dashboard" class="Bool (strict)"("DisabledEnum"=w1588) -> ()  [unwired: 2 in, 2 out]
        n1742 = property on="Analysis" class="Bool (strict)"("DisabledEnum"=w1588) -> ()  [unwired: 2 in, 2 out]
        n1743 = property on="Home" class="Bool (strict)"("DisabledEnum"=w1588) -> ()  [unwired: 2 in, 2 out]
        n1744 = property on="Report" class="Bool (strict)"("DisabledEnum"=w1588) -> ()  [unwired: 2 in, 2 out]
        n1745 = property on="Calibration" class="Bool (strict)"("DisabledEnum"=w1588) -> ()  [unwired: 2 in, 2 out]
      }
      frame "About" {
        n1746 = local read "FILE"() -> (w1607:string)
        n1747 = local read "TEST FILE NAM,E SAVED"() -> (w1600:bool)
        n1748 = call <vilib>:"Trim Whitespace.vi"("string"=w1607) -> ("trimmed string"=w1606:string)  [unwired: 1 in]
        n1749 = local read "Auto Start Test"() -> (w1610:bool)
        n1750 = String Length(string=w1606) -> (length=w1605:i32)
        n1751 = Greater?(x=w1605, y=1) -> (0:w1602:bool)
        n1752 = And(x=w1602, y=w1600) -> (x .and. y?=w1601:bool)
        n1753 = local read "RUN"() -> (w1612:bool)
        n1754 = case shown="True" w1601 {
          tunnel: [T19."Disabled" ("Disabled") T19."Enabled" ("Disabled")] -> w1603
          frame False {
          }
          frame True {
          }
        }
        n1755 = Or(x=w1612, y=w1610) -> (x .or. y?=w1611:bool)
        n1756 = property on="About" class="Bool (strict)"("DisabledEnum"=T19."Enabled" ("Disabled")) -> ()  [unwired: 2 in, 2 out]
        n1757 = case shown="False" w1611 {
          tunnel: [T19."Enabled" ("Disabled") T19."Disabled" ("Disabled")] -> w1609
          frame False {
          }
          frame True {
          }
        }
        n1758 = property on="Dashboard" class="Bool (strict)"("DisabledEnum"=w1603) -> ()  [unwired: 2 in, 2 out]
        n1759 = property on="Test Setup" class="Bool (strict)"("DisabledEnum"=T19."Disabled" ("Disabled")) -> ()  [unwired: 2 in, 2 out]
        n1760 = property on="Imaging" class="Bool (strict)"("DisabledEnum"=w1609) -> ()  [unwired: 2 in, 2 out]
        n1761 = property on="Analysis" class="Bool (strict)"("DisabledEnum"=w1609) -> ()  [unwired: 2 in, 2 out]
        n1762 = property on="Home" class="Bool (strict)"("DisabledEnum"=w1609) -> ()  [unwired: 2 in, 2 out]
        n1763 = property on="Report" class="Bool (strict)"("DisabledEnum"=w1609) -> ()  [unwired: 2 in, 2 out]
      }
    }
    n1764 = local read "Quit"() -> (w1537:bool)
    "Single" <- "Single - Graph"
  }
  n1765 = disable-structure shown="Disabled" {
    disable-tunnel: [w1890 _] -> w47
    disable-tunnel: _ -> [w1889 _]
    frame Disabled {
      n1766 = while {
        tunnel: w1889 -> [_]
        tunnel: [w1891] -> w1890
        tunnel: [w1892] -> _
        i -> [w1892]
        stop <- w1891 stop-if-true
        w1908 = u16 10 items=["1.0"=10, "1.5"=15, "2.0"=20] ("stop bits (10: 1 bit)")
        n1767 = Wait (ms)(milliseconds to wait=u32 10) -> ()  [unwired: 1 out]
        n1768 = call-poly "VISA Configure Serial Port"("VISA resource name"=refnum<visa-resource-name> "ASRL1::INSTR" ("COM PORT"), "timeout (10sec)"=u32 10, "baud rate (9600)"=u32 57600, "data bits (8)"=u16 8, "stop bits (10: 1 bit)"=w1908) -> ("VISA resource name out"=w1894:refnum<visa-resource-name>, "error out"=w1903:errorcluster)  [unwired: 9 in]
        n1769 = VISA Read(VISA resource name=w1894, byte count=u32 2 ("byte count (0)")) -> (read buffer=w1902:string)  [unwired: 1 in, 3 out]
        n1770 = String Subset(string=w1902, offset (0)=0, length (rest)=2 ("length (rest)")) -> (substring=w1901:string)
        n1771 = Match Pattern(string=w1901, regular expression="<>") -> (offset past match=w1898:i32)  [unwired: 1 in, 3 out]
        n1772 = Greater Or Equal?(x=w1898, y=0) -> (x >= y?=w1893:bool)
        n1773 = case shown="True" w1893 {
          tunnel: w1894 -> [_ w1912]
          tunnel: w1903 -> [_ w1911]
          frame False {
          }
          frame True {
            n1774 = VISA Read(VISA resource name=w1912, byte count=u32 32 ("byte count (0)"), error in (no error)=w1911) -> (read buffer=w1910:string)  [unwired: 3 out]
            n1775 = String Subset(string=w1910, offset (0)=0, length (rest)=8 ("length (rest)")) -> (substring=w1914:string)
            n1776 = String Subset(string=w1910, offset (0)=8, length (rest)=8 ("length (rest)")) -> (substring=w1915:string)
            n1777 = Decimal String To Number(string=w1915) -> (number=w1922:i32)  [unwired: 2 in, 1 out]
            n1778 = Decimal String To Number(string=w1914) -> (number=w1918:i32)  [unwired: 2 in, 1 out]
            n1779 = Divide(x=w1922, y=10000) -> ()  [unwired: 1 out]
            n1780 = Divide(x=w1918, y=1000000) -> ()  [unwired: 1 out]
          }
        }
        n1781 = local read "Quit"() -> (w1891:bool)
      }
    }
    frame Enabled {
    }
  }
  n1782 = Tick Count (ms)() -> (millisecond timer value=w9:u32)
  n1783 = while {
    shift-right: [w1968] -> _
    shift-left: w11 -> [w1972]
    shift-right: [w1967] -> _
    shift-left: w10 -> [w1971]
    shift-right: [w1966] -> _
    shift-left: w11 -> [w1970]
    shift-right: [w1965] -> _
    shift-left: w10 -> [w1969]
    shift-right: [w1963] -> _
    shift-left: w9 -> [w1964]
    shift-right: [w1960] -> _
    shift-left: w8 -> [w1961]
    shift-right: [w1959] -> _
    shift-left: w8 -> [w1962]
    shift-right: [w1952] -> _
    shift-left: w8 -> [w1958]
    shift-right: [w1951] -> _
    shift-left: w8 -> [w1957]
    shift-right: [w1950] -> _
    shift-left: w8 -> [w1956]
    shift-right: [w1949] -> _
    shift-left: w8 -> [w1955]
    shift-right: [w1948] -> _
    shift-left: w8 -> [w1954]
    shift-right: [w1947] -> _
    shift-left: w8 -> [w1953]
    shift-right: [w1946] -> _
    shift-left: w8 -> [w1940]
    shift-right: [w1945] -> _
    shift-left: w8 -> [w1939]
    shift-right: [w1944] -> _
    shift-left: w8 -> [w1938]
    shift-right: [w1943] -> _
    shift-left: w8 -> [w1937]
    shift-right: [w1942] -> _
    shift-left: w8 -> [w1936]
    shift-right: [w1941] -> _
    shift-left: w8 -> [w1935]
    shift-right: [w1926] -> _
    shift-left: w8 -> [w1929]
    shift-right: [w1925] -> _
    shift-left: w8 -> [w1928]
    shift-right: [w1924] -> _
    shift-left: w8 -> [w1927]
    stop <- w1974 stop-if-true
    n1784 = local read "Read UNO"() -> (w1933:string)
    n1785 = local read "Error  2"() -> (w1973:errorcluster)
    n1786 = String Length(string=w1933) -> (length=w1932:i32)
    n1787 = call <vilib>:"Trim Whitespace.vi"("string"=w1933) -> ("trimmed string"=w1934:string)  [unwired: 1 in]
    n1788 = Greater Or Equal?(x=w1932, y=23) -> (x >= y?=w1930:bool)
    n1789 = case shown="No Error" w1973 {
      tunnel: w1972 -> [w2020 w2116]
      tunnel: w1971 -> [w2019 w2115]
      tunnel: w1970 -> [w2018 w2114]
      tunnel: w1969 -> [w2017 w2113]
      tunnel: [w2016 w2116] -> w1968
      tunnel: [w2015 w2115] -> w1967
      tunnel: [w2014 w2114] -> w1966
      tunnel: [w2013 w2113] -> w1965
      tunnel: w1964 -> [w2012 w2112]
      tunnel: [w2011 w2112] -> w1963
      tunnel: w1961 -> [w2010 w2111]
      tunnel: w1962 -> [w2009 w2110]
      tunnel: [w2008 w2111] -> w1960
      tunnel: [w2007 w2110] -> w1959
      tunnel: w1958 -> [w2006 w2109]
      tunnel: w1957 -> [w2005 w2108]
      tunnel: w1956 -> [w2004 w2107]
      tunnel: w1955 -> [w2003 w2106]
      tunnel: w1954 -> [w2002 w2105]
      tunnel: w1953 -> [w2001 w2104]
      tunnel: [w2000 w2109] -> w1952
      tunnel: [w1999 w2108] -> w1951
      tunnel: [w1998 w2107] -> w1950
      tunnel: [w1997 w2106] -> w1949
      tunnel: [w1996 w2105] -> w1948
      tunnel: [w1995 w2104] -> w1947
      tunnel: w1940 -> [w1994 w2103]
      tunnel: [w1993 w2103] -> w1946
      tunnel: [w1992 w2099] -> w1945
      tunnel: [w1991 w2098] -> w1944
      tunnel: [w1990 w2102] -> w1943
      tunnel: [w1989 w2101] -> w1942
      tunnel: [w1988 w2100] -> w1941
      tunnel: w1939 -> [w1987 w2102]
      tunnel: w1938 -> [w1986 w2101]
      tunnel: w1937 -> [w1985 w2100]
      tunnel: w1936 -> [w1984 w2099]
      tunnel: w1935 -> [w1983 w2098]
      tunnel: w1934 -> [w1982 _]
      tunnel: w1930 -> [w1981 _]
      tunnel: w1929 -> [w1980 w2097]
      tunnel: w1928 -> [w1979 w2096]
      tunnel: w1927 -> [w1978 w2095]
      tunnel: [w1977 w2097] -> w1926
      tunnel: [w1976 w2096] -> w1925
      tunnel: [w1975 w2095] -> w1924
      frame No Error {
        n1790 = case shown="True" w1981 {
          tunnel: w2020 -> [w2036 w2088]
          tunnel: w2019 -> [w2035 w2087]
          tunnel: w2018 -> [w2034 w2086]
          tunnel: w2017 -> [w2033 w2085]
          tunnel: [w2036 w2084] -> w2016
          tunnel: [w2035 w2083] -> w2015
          tunnel: [w2034 w2082] -> w2014
          tunnel: [w2033 w2081] -> w2013
          tunnel: w2012 -> [w2032 w2079]
          tunnel: [w2032 w2078] -> w2011
          tunnel: w2010 -> [w2031 w2077]
          tunnel: w2009 -> [w2030 w2076]
          tunnel: [w2031 w2075] -> w2008
          tunnel: [w2030 w2074] -> w2007
          tunnel: w2006 -> [w2029 w2073]
          tunnel: w2005 -> [w2028 w2072]
          tunnel: w2004 -> [w2027 w2071]
          tunnel: w2003 -> [w2026 w2070]
          tunnel: w2002 -> [w2025 w2069]
          tunnel: w2001 -> [w2024 w2068]
          tunnel: [w2029 w2067] -> w2000
          tunnel: [w2028 w2066] -> w1999
          tunnel: [w2027 w2065] -> w1998
          tunnel: [w2026 w2064] -> w1997
          tunnel: [w2025 w2063] -> w1996
          tunnel: [w2024 w2062] -> w1995
          tunnel: w1994 -> [w2042 w2061]
          tunnel: [w2042 w2060] -> w1993
          tunnel: [w2039 w2059] -> w1992
          tunnel: [w2038 w2058] -> w1991
          tunnel: [w2041 w2057] -> w1990
          tunnel: [w2037 w2056] -> w1989
          tunnel: [w2040 w2055] -> w1988
          tunnel: w1987 -> [w2041 w2054]
          tunnel: w1986 -> [w2040 w2053]
          tunnel: w1985 -> [w2039 w2052]
          tunnel: w1984 -> [w2038 w2051]
          tunnel: w1983 -> [w2037 w2050]
          tunnel: w1982 -> [_ w2049]
          tunnel: w1980 -> [w2023 w2048]
          tunnel: w1979 -> [w2022 w2047]
          tunnel: w1978 -> [w2021 w2046]
          tunnel: [w2023 w2045] -> w1977
          tunnel: [w2022 w2044] -> w1976
          tunnel: [w2021 w2043] -> w1975
          frame False {
          }
          frame True {
            n1791 = Tick Count (ms)() -> (millisecond timer value=w2080:u32)
            n1792 = String To Byte Array(string=w2049) -> (unsigned byte array=w2093:u8[])
            n1793 = Array Size(array=w2093) -> (size(s)=w2092:i32)
            n1794 = formula code="// --- INTERNAL VARIABLE DECLARATIONS ---\nint i = 0;\nint k = 0;\nint start_idx = -1;\nint end_idx = -1;\nint phase = 0;\nint sign0 = 1;\nint sign1 = 1;\nint ch0_val = 0;   \nint ch1_val = 0;   \nfloat ch0_raw = 0.0;\nfloat ch1_raw = 0.0;\nfloat temp0 = 0.0;\nfloat temp1 = 0.0;\nfloat ch0_clean = 0.0;\nfloat ch1_clean = 0.0;\n\nint valid_samples = 0; // FIX: Track if we actually parsed new data this window\nfloat max_allowed_bits = 8388607.0; // FIX: Change this to match your ADC max value\n\n// Temporal intermediate variables for calculation smoothing\nfloat raw_p2p_v = 0.0;\nfloat raw_friction = 0.0;\nfloat raw_cof = 0.0;\n\n// Temporal intermediate variables for Piezo voltage translations\nfloat piezo_min_v = 0.0;\nfloat piezo_max_v = 0.0;\n\n// Initialize output variables to current shift register states right away\nout_LVDT_Min_V = in_LVDT_Min_V;\nout_LVDT_Max_V = in_LVDT_Max_V;\nout_LVDT_P2P_V = in_LVDT_P2P_V;\nout_Piezo_P2P = in_Piezo_P2P;\nout_Friction_N = in_Friction_N;\nout_COF = in_COF;\nwindow_ready = 0;\n\n// --- STEP 1: PARSE EVERY STRING IN THE BYTE ARRAY ---\nif (array_size > 2) {\n    for (i = 0; i < array_size - 1; i++) {\n        if (raw_bytes[i] == 42) { // '*' character detected\n            start_idx = i;\n        }\n        \n        // Match standard delimiter sequence \";&\" or end window character\n        if (raw_bytes[i] == 59 && raw_bytes[i+1] == 38 && start_idx != -1) { \n            end_idx = i;\n            ch0_val = 0;\n            ch1_val = 0;\n            sign0 = 1;\n            sign1 = 1;\n            phase = 0; \n\n            for (k = start_idx + 1; k < end_idx; k++) {\n                if (raw_bytes[k] == 45) { // '-' sign\n                    if (phase == 0) sign0 = -1;\n                    else sign1 = -1;\n                }\n                else if (raw_bytes[k] == 43) { // '+' sign\n                    if (phase == 0) sign0 = 1;\n                    else sign1 = 1;\n                }\n                else if (raw_bytes[k] == 59) { // ';' delimiter\n                    phase = 1; \n                }\n                else if (raw_bytes[k] >= 48 && raw_bytes[k] <= 57) { // Numeric ASCII digits\n                    if (phase == 0) {\n                        ch0_val = (ch0_val * 10) + (raw_bytes[k] - 48);\n                    } else {\n                        ch1_val = (ch1_val * 10) + (raw_bytes[k] - 48);\n                    }\n                }\n            }\n\n            // Implicit type conversion\n            ch0_raw = ch0_val * sign0 * 1.0;\n            ch1_raw = ch1_val * sign1 * 1.0;\n\n            // FIX: Sanity check / Hard-clamping to catch sudden massive ASCII noise spikes\n            if (ch0_raw > max_allowed_bits)  ch0_raw = max_allowed_bits;\n            if (ch0_raw < -max_allowed_bits) ch0_raw = -max_allowed_bits;\n            if (ch1_raw > max_allowed_bits)  ch1_raw = max_allowed_bits;\n            if (ch1_raw < -max_allowed_bits) ch1_raw = -max_allowed_bits;\n\n            // --- STEP 2: 3-SAMPLE MEDIAN FILTER ---\n            m0_2 = m0_1; m0_1 = m0_0; m0_0 = ch0_raw;\n            float s0_0 = m0_0; float s0_1 = m0_1; float s0_2 = m0_2;\n            if (s0_0 > s0_1) { temp0 = s0_0; s0_0 = s0_1; s0_1 = temp0; }\n            if (s0_1 > s0_2) { temp0 = s0_1; s0_1 = s0_2; s0_2 = temp0; }\n            if (s0_0 > s0_1) { temp0 = s0_0; s0_0 = s0_1; s0_1 = temp0; }\n            ch0_clean = s0_1;\n\n            m1_2 = m1_1; m1_1 = m1_0; m1_0 = ch1_raw;\n            float s1_0 = m1_0; float s1_1 = m1_1; float s1_2 = m1_2;\n            if (s1_0 > s1_1) { temp1 = s1_0; s1_0 = s1_1; s1_1 = temp1; }\n            if (s1_1 > s1_2) { temp1 = s1_1; s1_1 = s1_2; s1_2 = temp1; }\n            if (s1_0 > s1_1) { temp1 = s1_0; s1_0 = s1_1; s1_1 = temp1; }\n            ch1_clean = s1_1;\n\n            // --- STEP 3: EXPONENTIAL FILTER (STREAM LEVEL) ---\n            if (ch0_filt == 0.0) ch0_filt = ch0_clean;\n            if (ch1_filt == 0.0) ch1_filt = ch1_clean;\n\n            ch0_filt = ch0_filt + (ch0_clean - ch0_filt) * 0.125;\n            ch1_filt = ch1_filt + (ch1_clean - ch1_filt) * 0.125;\n\n            // --- STEP 4: MIN/MAX WINDOW CONTINUOUS ACCUMULATION ---\n            if (ch0_filt > max_ch0) max_ch0 = ch0_filt;\n            if (ch0_filt < min_ch0) min_ch0 = ch0_filt;\n            if (ch1_filt > max_ch1) max_ch1 = ch1_filt;\n            if (ch1_filt < min_ch1) min_ch1 = ch1_filt;\n\n            valid_samples++; // FIX: Successfully parsed and accumulated a clean point\n            start_idx = -1; \n        }\n    }\n}\n\n// --- STEP 5: WINDOW EVALUATION ENGINE ---\n// FIX: Condition updated to verify that valid samples exist for both channels\nif (((current_time_ms - start_time_ms) >= 50) && (valid_samples > 0) && (min_ch0 < 9000000.0) && (min_ch1 < 9000000.0)) {\n    window_ready = 1;\n\n    // Linear Bit-to-Voltage Transformations (LVDT - Channel 0)\n    out_LVDT_Min_V = (min_ch0 * VREF) / 8388607.0;\n    out_LVDT_Max_V = (max_ch0 * VREF) / 8388607.0;\n    raw_p2p_v = out_LVDT_Max_V - out_LVDT_Min_V;\n\n    // Linear Bit-to-Voltage Transformations (Piezo - Channel 1)\n    piezo_min_v = (min_ch1 * VREF) / 8388607.0;\n    piezo_max_v = (max_ch1 * VREF) / 8388607.0;\n    \n    // Assign Peak-to-Peak Voltage directly to output indicator (Matches Python logic)\n    out_Piezo_P2P = piezo_max_v - piezo_min_v;\n    \n    // Force scaling calculations using Voltage delta * Newtons/Volt Factor\n    raw_friction = out_Piezo_P2P * PIEZO_CAL_FACTOR ;\n    raw_cof = raw_friction / NORMAL_FORCE;\n\n    // --- STEP 6: OUTPUT METRIC SMOOTHING (Low-Pass Filter Alpha = 0.05) ---\n    // Seed initial historical metrics if first loop iteration\n    if (hist_LVDT_P2P == 0.0) hist_LVDT_P2P = raw_p2p_v;\n    if (hist_Friction == 0.0) hist_Friction = raw_friction;\n    if (hist_COF == 0.0)      hist_COF = raw_cof;\n\n    // Apply exponential output dampening\n    hist_LVDT_P2P = hist_LVDT_P2P + (raw_p2p_v - hist_LVDT_P2P) * 0.05;\n    hist_Friction = hist_Friction + (raw_friction - hist_Friction) * 0.05; // Note: Can drop to 0.02 for more aggressive damping\n    hist_COF      = hist_COF + (raw_cof - hist_COF) * 0.05;\n\n    // Direct smoothed parameters out to UI Indicators\n    out_LVDT_P2P_V = hist_LVDT_P2P;\n    out_Friction_N = hist_Friction;\n    out_COF        = hist_COF;\n\n    // Reset tracking targets to extreme boundaries safely\n    min_ch0 = 9999999.0;\n    max_ch0 = -9999999.0;\n    min_ch1 = 9999999.0;\n    max_ch1 = -9999999.0;\n\n    valid_samples = 0; // FIX: Reset counter for next time frame\n    start_time_ms = current_time_ms;\n}"("raw_bytes"=w2093, "array_size"=w2092, "VREF"="VREF", "PIEZO_CAL_FACTOR"="PIEZO_CAL_FACTOR", "NORMAL_FORCE"="NORMAL_FORCE", "min_ch0"=w2088, "max_ch0"=w2087, "min_ch1"=w2086, "max_ch1"=w2085, "current_time_ms"=w2080, "start_time_ms"=w2079, "ch0_filt"=w2077, "ch1_filt"=w2076, "m0_0"=w2073, "m0_1"=w2072, "m0_2"=w2071, "m1_0"=w2070, "m1_1"=w2069, "m1_2"=w2068, "in_LVDT_Min_V"=w2061, "in_LVDT_Max_V"=w2054, "in_LVDT_P2P_V"=w2053, "in_Piezo_P2P"=w2052, "in_Friction_N"=w2051, "in_COF"=w2050, "hist_LVDT_P2P"=w2048, "hist_Friction"=w2047, "hist_COF"=w2046) -> ("window_ready"=→"Valid_data":dbl, "out_LVDT_Min_V"=w2060:dbl, "out_LVDT_Max_V"=w2059:dbl, "out_LVDT_P2P_V"=w2058:dbl, "out_Piezo_P2P"=w2057:dbl, "out_Friction_N"=w2056:dbl, "out_COF"=w2055:dbl, "min_ch0"=w2084:dbl, "max_ch0"=w2083:dbl, "min_ch1"=w2082:dbl, "max_ch1"=w2081:dbl, "start_time_ms"=w2078:u32, "ch0_filt"=w2075:dbl, "ch1_filt"=w2074:dbl, "m0_0"=w2067:dbl, "m0_1"=w2066:dbl, "m0_2"=w2065:dbl, "m1_0"=w2064:dbl, "m1_1"=w2063:dbl, "m1_2"=w2062:dbl, "hist_LVDT_P2P"=w2045:dbl, "hist_Friction"=w2044:dbl, "hist_COF"=w2043:dbl)